vi "Button and Switch CCS.vi"() -> ()   [LabVIEW 2020]
uses:
  <vilib>/addons/control/pid/autopid.llb/PID autotuning parameters (adv).ctl
  <vilib>/addons/control/pid/pid.llb/PID Time Unit.ctl
  <vilib>/addons/control/pid/pid.llb/PID Structure.ctl
  <vilib>/addons/control/pid/pid.llb/PID Gain Unit.ctl
  <vilib>/Instr/_visa.llb/VISA Configure Serial Port (Instr).vi
  <vilib>/addons/control/pid/pid.llb/PID Structure Conversion (DBL).vi
  <vilib>/addons/control/pid/pid.llb/PID Advanced (DBL).vi
  <vilib>/addons/control/pid/NI_PID_autopid.lvlib
  <vilib>/ptbypt/NI_PtbyPt.lvlib
  <vilib>/addons/control/pid/NI_PID_pid.lvlib
panel:
  out "Image Out 2":T1(plugin-control) caption="Image Out"
  out "D":bool
  out "N":bool=TRUE
  out "R":bool
  out "P":bool
  out "PWM Previous":dbl
  in  "auto? ACC":bool
  out "Limit Setpoint":u64
  out "Limit Active":bool
  in  "Limit -":bool
  in  "Limit +":bool
  in  "Limit Speed":bool
  in  "gamma":dbl format="%.2f"
  in  "alpha":dbl=0.2 format="%.2f"
  in  "proportional unit":T2 items=["Gain (K)", "Band (PB)"]
  in  "PID structure":T3 items=["Academic (Standard)", "Parallel", "Series"]
  in  "derivative unit":T4=1 items=["min", "s"]
  in  "integral unit":T4=1 items=["min", "s"]
  in  "derivative":dbl
  in  "integral":dbl
  in  "proportional":dbl=10.0
  in  "linearity":dbl=0.9 format="%.2f"
  in  "beta":dbl=0.7 format="%.2f"
  in  "reinitialize? (F) 2":bool
  out "Speed Setpoint (km/h)":dbl
  out "Target Distance (m)":dbl
  out "Time Level":dbl=2.1
  out "Distance (m)":i8=66
  out "Brake Light":bool
  in  "VISA resource name":refnum<visa-resource-name>="COM5"
  in  "baud rate":u32=115200
  out "RPM":i64(knob) scale=0.0..650.0
  out "VELOCITY":u64(knob) scale=0.0..200.0
  out "GAS PEDAL":u8(slide) scale=0.0..255.0
  out "BRAKE PEDAL":u8(slide) scale=0.0..255.0
  out "VELOCITY":cluster{"VELOCITY":u64, "Cruise Setpoint":u64}(graph)
  in  "autotune? (F)":bool
  in  "PID gains":T5={"proportional gain (Kc)"=0.261831, "integral time (Ti, min)"=0.013639, "derivative time (Td, min)"=0.0} {"derivative time (Td, min)" format="%#.6g"; "integral time (Ti, min)" format="%#.6g"; "proportional gain (Kc)" format="%#.6g"}
  in  "dt (s)":dbl=0.02
  in  "reinitialize? (F)":bool
  in  "autotuning parameters":T6={"technique"=0, "type of controller"=1, "control specification"=0, "amplitude"=30.0} {"amplitude" format="%.2f"; "control specification" items=["normal", "fast", "slow"]; "type of controller" items=["P", "PI", "PID"]; "technique" items=["Step Open Loop", "Step Closed Loop", "Relay", "PID Relay"]}
  out "completed?":bool
  out "tuned PID gains":T5={"proportional gain (Kc)"=0.261831, "integral time (Ti, min)"=0.013639, "derivative time (Td, min)"=0.0} {"derivative time (Td, min)" format="%#.6g"; "integral time (Ti, min)" format="%#.6g"; "proportional gain (Kc)" format="%#.6g"}
  in  "auto? Speed Control":bool
  in  "ACCEPT SPEED PID":bool
  out "MOTOR CONTROL":dbl(graph)
  in  "stop":bool
  in  "PID Mode":i64(knob)=1 scale=1.0..3.0
  in  "Cruise Enable":bool
  in  "Distance":bool
  out "Distance Level":i8=4
  out "Cruise Active":bool
  out "Cruise Setpoint":u64
  in  "Speed +":bool
  in  "Speed -":bool
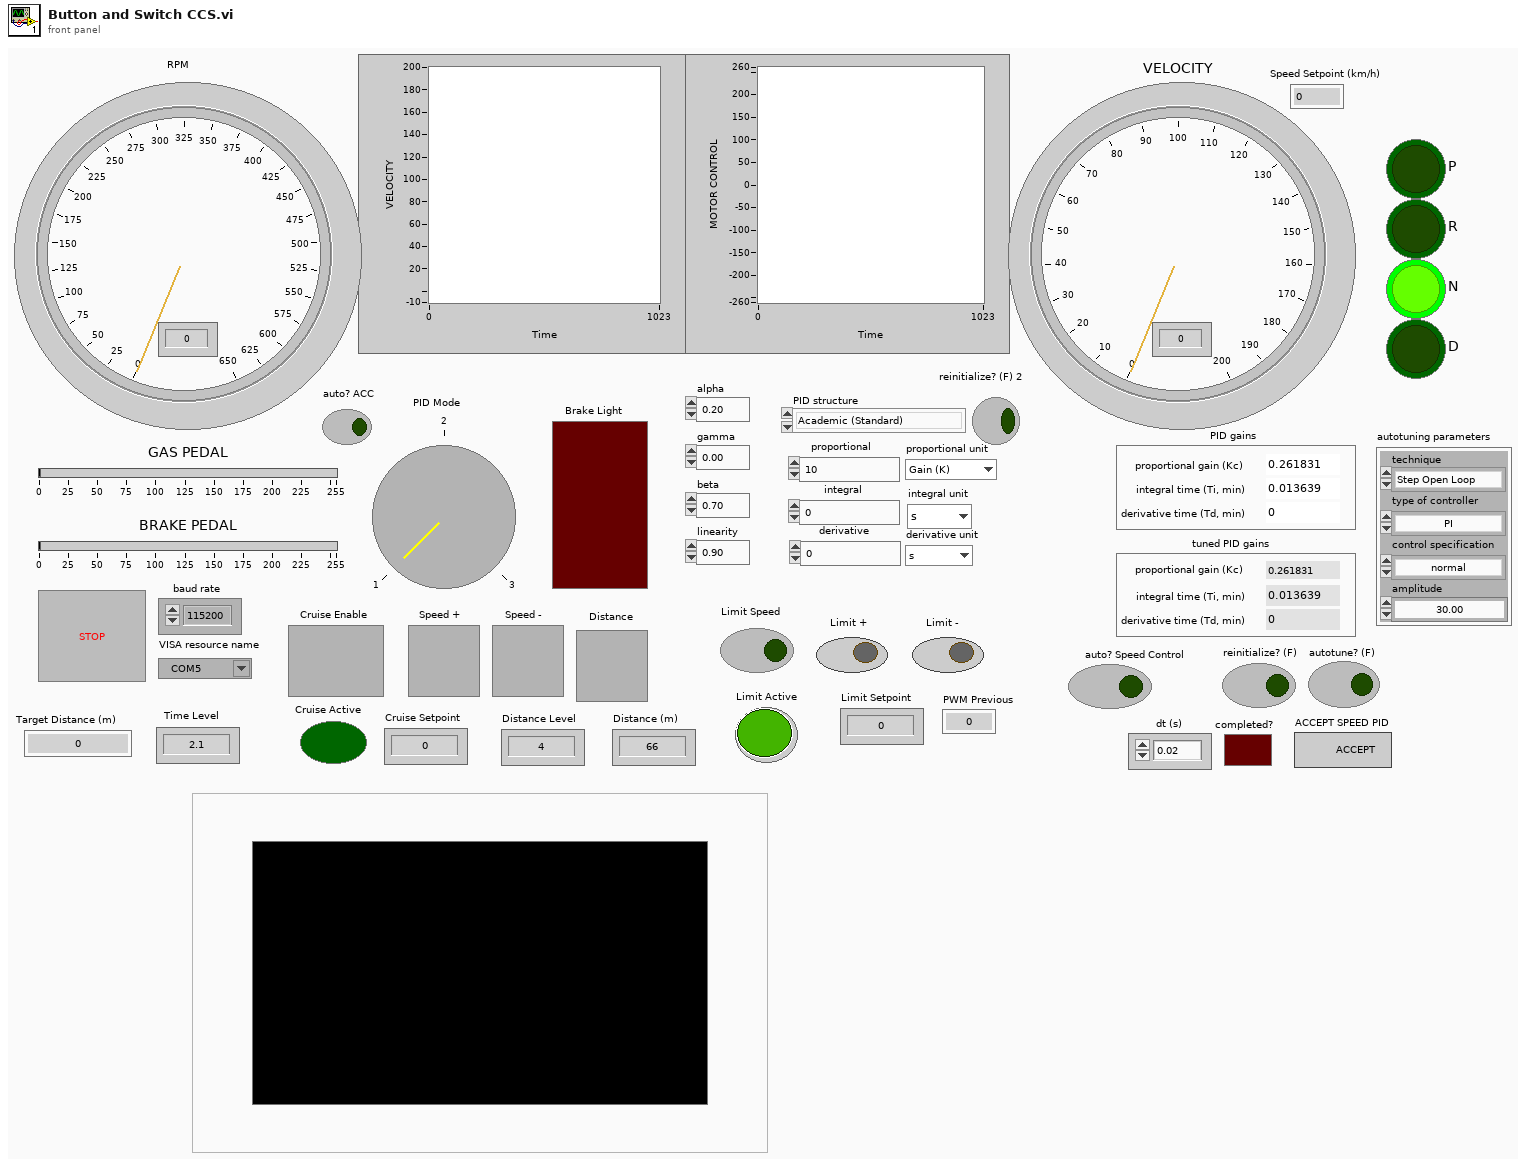
[diagram p1: front panel]
types:
  T1 = typedef "IMAQ Image.ctl" = refnum<image>
  T2 = typedef "NI_PID_pid.lvlib/PID Gain Unit.ctl" = u16
  T3 = typedef "NI_PID_pid.lvlib/PID Structure.ctl" = u16
  T4 = typedef "NI_PID_pid.lvlib/PID Time Unit.ctl" = u16
  T5 = cluster{"proportional gain (Kc)":dbl, "integral time (Ti, min)":dbl, "derivative time (Td, min)":dbl}
  T6 = typedef "NI_PID_autopid.lvlib/PID autotuning parameters (adv).ctl" = cluster{"technique":u16, "type of controller":u16, "control specification":u16, "amplitude":dbl}
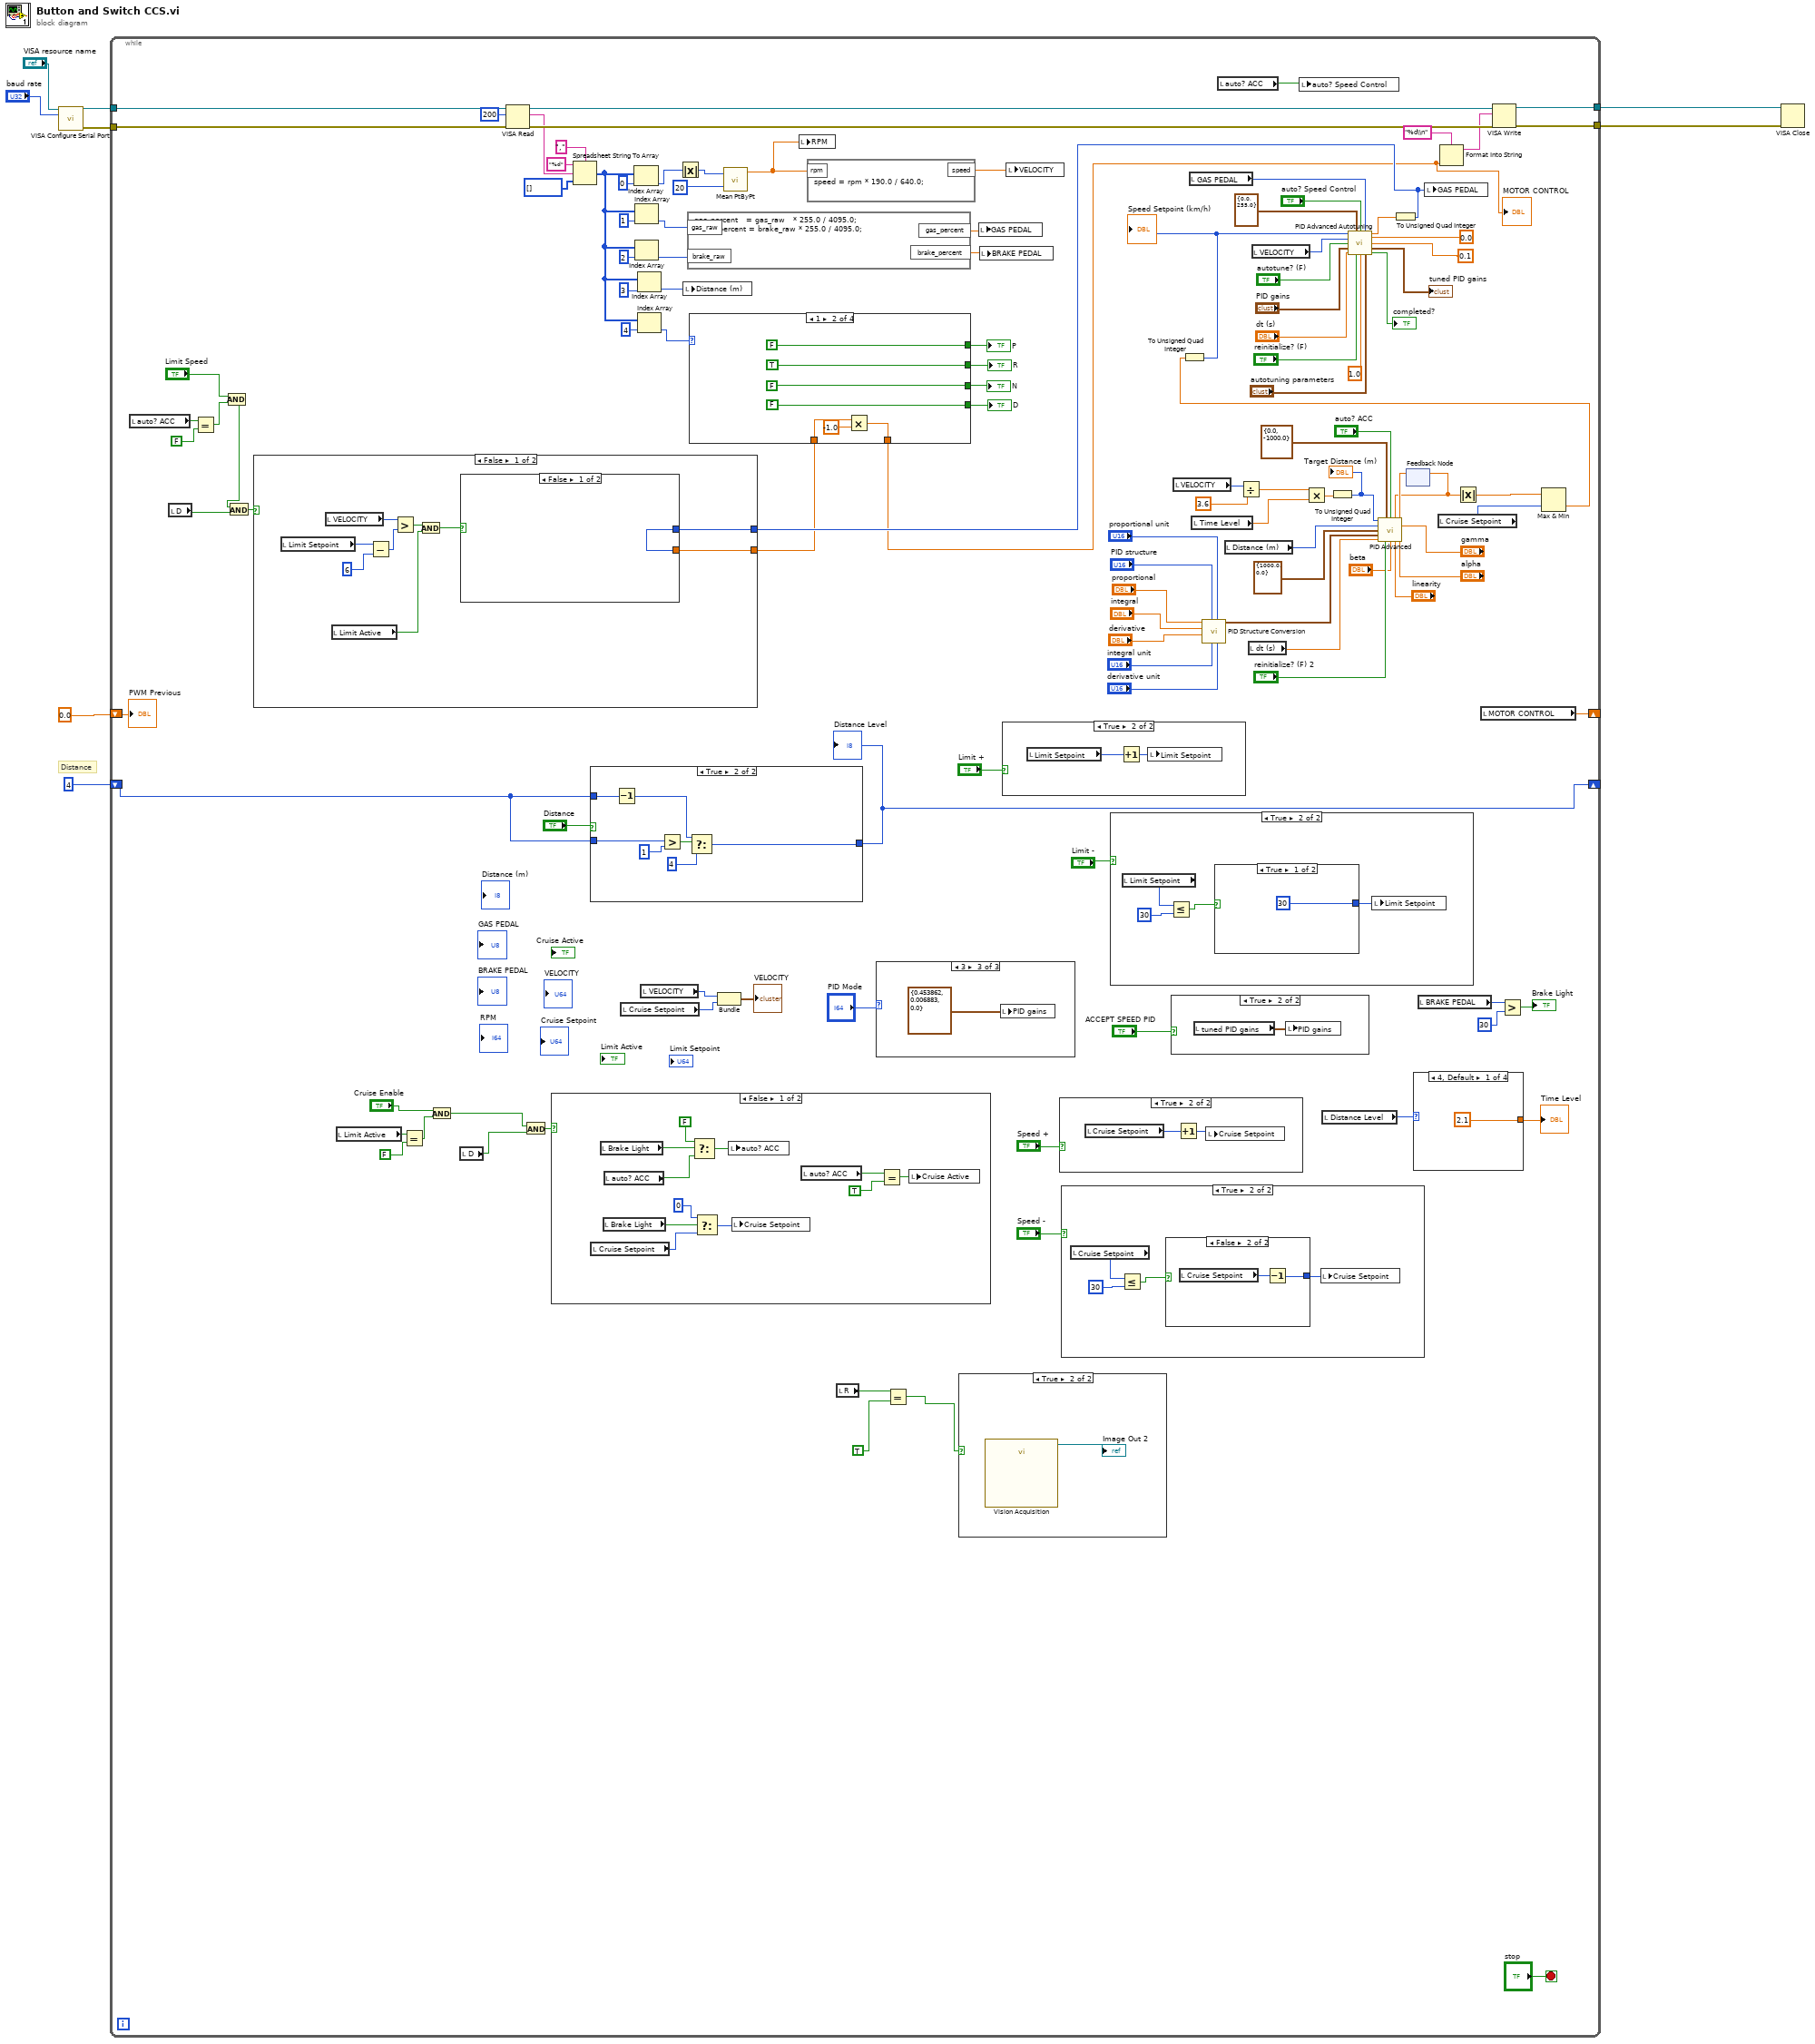
[diagram p0: block diagram]
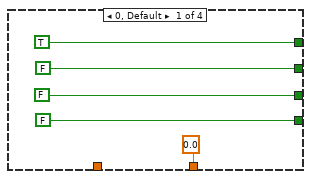
[diagram p3: hidden frame]
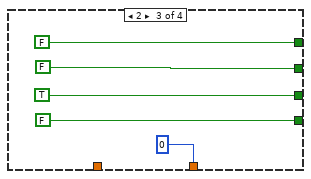
[diagram p4: hidden frame]
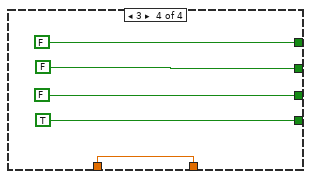
[diagram p5: hidden frame]
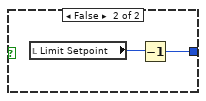
[diagram p7: hidden frame]
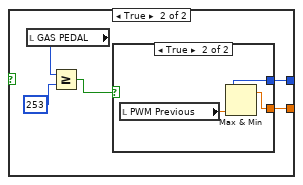
[diagram p9: hidden frame]
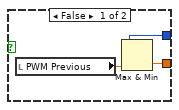
[diagram p10: hidden frame]
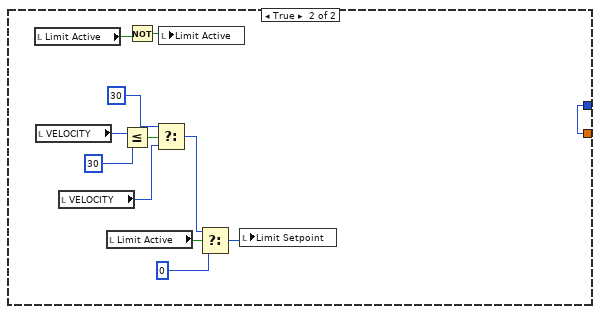
[diagram p11: hidden frame]
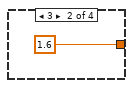
[diagram p12: hidden frame]
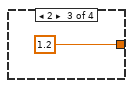
[diagram p13: hidden frame]
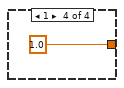
[diagram p14: hidden frame]
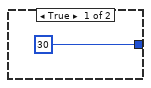
[diagram p17: hidden frame]
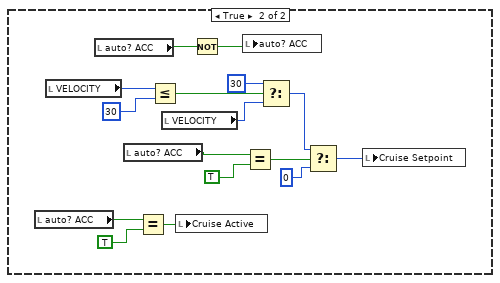
[diagram p19: hidden frame]
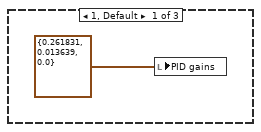
[diagram p20: hidden frame]
diagram:
  # "Distance"
  n1 = call-poly "VISA Configure Serial Port"("VISA resource name"="VISA resource name", "baud rate (9600)"="baud rate") -> ("VISA resource name out"=w7:refnum<visa-resource-name>, "error out"=w6:errorcluster)  [unwired: 12 in]
  n2 = while {
    tunnel: w7 -> [w128]
    tunnel: w6 -> [w127]
    tunnel: [w102] -> w5
    tunnel: [w103] -> w4
    shift-right: [w80] -> _
    shift-left: i64 4 ("f") -> [w81]
    shift-right: [w37] -> _
    shift-left: 0.0 ("MOTOR CONTROL") -> [w35]
    stop <- "stop" stop-if-true
    n3 = local read "auto? ACC"() -> (w41:bool)
    n4 = local read "D"() -> (w17:bool)
    n5 = Equal?(x=w41, y=FALSE) -> (x = y?=w40:bool)
    n6 = And(x="Limit Speed", y=w40) -> (x .and. y?=w18:bool)
    n7 = And(x=w18, y=w17) -> (x .and. y?=w19:bool)
    n8 = local read "Limit Active"() -> (w31:bool)
    n9 = Equal?(x=w31, y=FALSE) -> (x = y?=w32:bool)
    n10 = And(x="Cruise Enable", y=w32) -> (x .and. y?=w15:bool)
    n11 = local read "D"() -> (w14:bool)
    n12 = VISA Read(VISA resource name=w128, byte count=u32 200, error in (no error)=w127) -> (VISA resource name out=w125:refnum<visa-resource-name>, read buffer=w123:string, error out=w126:errorcluster)  [unwired: 1 out]
    n13 = And(x=w15, y=w14) -> (x .and. y?=w16:bool)
    n14 = case shown="False" w16 {
      frame False {
        n15 = local read "Cruise Setpoint"() -> (w217:u64)
        n16 = local read "Brake Light"() -> (w225:bool)
        n17 = local read "Brake Light"() -> (w218:bool)
        n18 = local read "auto? ACC"() -> (w222:bool)
        n19 = Select(t=FALSE, s=w225, f=w222) -> (s? t:f=w223:bool)
        n20 = Select(t=u64 0, s=w218, f=w217) -> (s? t:f=w215:u64)
        n21 = local write "auto? ACC"(w223) -> ()
        n22 = local write "Cruise Setpoint"(w215) -> ()
        n23 = local read "auto? ACC"() -> (w220:bool)
        n24 = Equal?(x=w220, y=TRUE) -> (x = y?=w219:bool)
        n25 = local write "Cruise Active"(w219) -> ()
      }
      frame True {
        n26 = local read "auto? ACC"() -> (w233:bool)
        n27 = local read "VELOCITY"() -> (w232:u64)
        n28 = local read "auto? ACC"() -> (w241:bool)
        n29 = local read "auto? ACC"() -> (w239:bool)
        n30 = Equal?(x=w233, y=TRUE) -> (x = y?=w226:bool)
        n31 = Less Or Equal?(x=w232, y=u64 30) -> (x <= y?=w230:bool)
        n32 = local read "VELOCITY"() -> (w229:u64)
        n33 = local write "Cruise Active"(w226) -> ()
        n34 = Not(x=w241) -> (.not. x?=w240:bool)
        n35 = local write "auto? ACC"(w240) -> ()
        n36 = Equal?(x=w239, y=TRUE) -> (x = y?=w237:bool)
        n37 = Select(t=u64 30, s=w230, f=w229) -> (s? t:f=w227:u64)
        n38 = Select(t=w227, s=w237, f=i64 0) -> (s? t:f=w236:u64)
        n39 = local write "Cruise Setpoint"(w236) -> ()
      }
    }
    n40 = Spreadsheet String To Array(delimiter (Tab)=",", format string="%d", spreadsheet string=w123, array type (2D Dbl)=i32[] []) -> (array=w26:i32[])
    n41 = case shown="True" "Distance" {
      tunnel: w81 -> [w198 w205]
      tunnel: w81 -> [_ w204]
      tunnel: [w198 w199] -> w80
      frame False {
      }
      frame True {
        n42 = Decrement(x=w205) -> (x-1=w201:i64)
        n43 = Greater?(x=w204, y=i64 1) -> (0:w202:bool)
        n44 = Select(t=w201, s=w202, f=i64 4) -> (s? t:f=w199:i64)
      }
    }
    "Distance Level" <- w80
    n45 = local read "Cruise Setpoint"() -> (w85:u64)
    n46 = Index Array(array=w26, index=0) -> (element=w96:i32)
    n47 = Index Array(array=w26, index=1) -> (element=w99:i32)
    n48 = Index Array(array=w26, index=2) -> (element=w98:i32)
    n49 = Index Array(array=w26, index=3) -> (element=w75:i32)
    n50 = Index Array(array=w26, index=4) -> (element=w24:i32)
    n51 = local read "VELOCITY"() -> (w91:u64)
    n52 = Absolute Value(x=w96) -> (abs(x)=w95:i32)
    n53 = local write "Distance (m)"(w75) -> ()
    n54 = formula code="gas_percent   = gas_raw   * 255.0 / 4095.0;\nbrake_percent = brake_raw * 255.0 / 4095.0;"("gas_raw"=w99, "brake_raw"=w98) -> ("gas_percent"=w34:dbl, "brake_percent"=w97:dbl)
    n55 = Bundle("VELOCITY"=w91, "Cruise Setpoint"=w85) -> (→"VELOCITY":cluster{"VELOCITY":u64, "Cruise Setpoint":u64})  [unwired: 1 in]
    n56 = call <vilib>:"Mean PtByPt.vi"("x"=w95, "sample length"=20) -> ("mean"=w100:dbl)  [unwired: 2 in, 1 out]
    n57 = local write "RPM"(w100) -> ()
    n58 = formula code="speed = rpm * 190.0 / 640.0;"("rpm"=w100) -> ("speed"=w101:dbl)
    n59 = local read "R"() -> (w11:bool)
    n60 = case shown="3" "PID Mode" {
      frame 1, Default {
        n61 = local write "PID gains"(T5 {"proportional gain (Kc)"=0.261831, "integral time (Ti, min)"=0.013639, "derivative time (Td, min)"=0.0} ("PID gains")) -> ()
      }
      frame 2 {
        n62 = local write "PID gains"(T5 {"proportional gain (Kc)"=0.638776, "integral time (Ti, min)"=0.011721, "derivative time (Td, min)"=0.0} ("PID gains")) -> ()
      }
      frame 3 {
        n63 = local write "PID gains"(T5 {"proportional gain (Kc)"=0.453862, "integral time (Ti, min)"=0.006883, "derivative time (Td, min)"=0.0} ("PID gains")) -> ()
      }
    }
    n64 = Equal?(x=w11, y=TRUE) -> (x = y?=w9:bool)
    n65 = case shown="True" w9 {
      frame False {
      }
      frame True {
        n66 = call "Vision Acquisition"() -> ("Image Out"=→"Image Out 2":T1)  [unwired: 23 in, 4 out]
      }
    }
    n67 = local write "GAS PEDAL"(w34) -> ()
    n68 = local write "BRAKE PEDAL"(w97) -> ()
    n69 = case shown="True" "Limit +" {
      frame False {
      }
      frame True {
        n70 = local read "Limit Setpoint"() -> (w160:u64)
        n71 = Increment(x=w160) -> (x+1=w159:u64)
        n72 = local write "Limit Setpoint"(w159) -> ()
      }
    }
    n73 = local write "VELOCITY"(w101) -> ()
    n74 = case shown="True" "Speed +" {
      frame False {
      }
      frame True {
        n75 = local read "Cruise Setpoint"() -> (w213:u64)
        n76 = Increment(x=w213) -> (x+1=w214:u64)
        n77 = local write "Cruise Setpoint"(w214) -> ()
      }
    }
    n78 = case shown="True" "Speed -" {
      frame False {
      }
      frame True {
        n79 = local read "Cruise Setpoint"() -> (w208:u64)
        n80 = Less Or Equal?(x=w208, y=u64 30) -> (x <= y?=w206:bool)
        n81 = case shown="False" w206 {
          tunnel: [u64 30 ("y") w211] -> w209
          frame True {
          }
          frame False {
            n82 = local read "Cruise Setpoint"() -> (w212:u64)
            n83 = Decrement(x=w212) -> (x-1=w211:u64)
          }
        }
        n84 = local write "Cruise Setpoint"(w209) -> ()
      }
    }
    n85 = case shown="True" "Limit -" {
      frame False {
      }
      frame True {
        n86 = local read "Limit Setpoint"() -> (w154:u64)
        n87 = Less Or Equal?(x=w154, y=u64 30) -> (x <= y?=w152:bool)
        n88 = case shown="True" w152 {
          tunnel: [u64 30 ("y") w157] -> w155
          frame True {
          }
          frame False {
            n89 = local read "Limit Setpoint"() -> (w158:u64)
            n90 = Decrement(x=w158) -> (x-1=w157:u64)
          }
        }
        n91 = local write "Limit Setpoint"(w155) -> ()
      }
    }
    n92 = case shown="True" "ACCEPT SPEED PID" {
      frame False {
      }
      frame True {
        n93 = local read "tuned PID gains"() -> (w245:T5)
        n94 = local write "PID gains"(w245) -> ()
      }
    }
    n95 = local read "VELOCITY"() -> (w69:u64)
    n96 = local read "GAS PEDAL"() -> (w86:u8)
    n97 = local read "Time Level"() -> (w70:dbl)
    n98 = call-poly <vilib>:"PID Structure Conversion.vi"("derivative unit"="derivative unit", "proportional unit"="proportional unit", "integral unit"="integral unit", "PID structure"="PID structure", "derivative"="derivative", "integral"="integral", "proportional"="proportional") -> ("PID gains"=w46:T5)  [unwired: 4 in]
    n99 = local read "auto? ACC"() -> (w42:bool)
    n100 = local read "Distance (m)"() -> (w68:i8)
    n101 = Divide(x=w69, y=3.6) -> (x/y=w71:dbl)
    n102 = local read "dt (s)"() -> (w62:dbl)
    n103 = local read "VELOCITY"() -> (w114:u64)
    n104 = local write "auto? Speed Control"(w42) -> ()
    n105 = Multiply(x=w71, y=w70) -> (x*y=w57:dbl)
    n106 = local read "Distance Level"() -> (w74:i8)
    n107 = To Unsigned Quad Integer(1:w57) -> (0:w56:u64)
    "Target Distance (m)" <- w56
    n108 = feedback #1() -> (w61:dbl)  [unwired: 1 in]
    n109 = call-poly <vilib>:"PID Advanced.vi"("setpoint"=w56, "output range"=cluster{"output high":dbl, "output low":dbl} {"output high"=0.0, "output low"=-1000.0}, "auto? (T)"="auto? ACC", "manual control"=w61, "process variable"=w68, "gamma"="gamma", "setpoint range"=cluster{"setpoint high":dbl, "setpoint low":dbl} {"setpoint high"=1000.0, "setpoint low"=0.0}, "alpha"="alpha", "PID gains"=w46, "dt (s)"=w62, "reinitialize? (F)"="reinitialize? (F) 2", "beta"="beta", "linearity"="linearity") -> ("output"=w63:dbl)  [unwired: 1 in, 1 out]
    n110 = feedback-in #1(w63) -> ()
    n111 = case shown="4, Default" w74 {
      tunnel: [2.1 ("Time Level") 1.6 ("Time Level") 1.2 ("Time Level") 1.0 ("Time Level")] -> w73
      frame 4, Default {
      }
      frame 3 {
      }
      frame 2 {
      }
      frame 1 {
      }
    }
    "Time Level" <- w73
    n112 = local read "BRAKE PEDAL"() -> (w79:u8)
    n113 = local read "Cruise Setpoint"() -> (w65:u64)
    n114 = Absolute Value(x=w61) -> (abs(x)=w60:dbl)
    n115 = local read "MOTOR CONTROL"() -> (w37:dbl)
    n116 = Greater?(x=w79, y=u8 30) -> (0:→"Brake Light":bool)
    n117 = Max & Min(x=w60, y=w65) -> (min(x,y)=w54:dbl)  [unwired: 1 out]
    n118 = To Unsigned Quad Integer(1:w54) -> (0:w55:u64)
    "Speed Setpoint (km/h)" <- w55
    n119 = call <vilib>:"PID Advanced Autotuning.vi"("setpoint"=w55, "output range"=cluster{"output high":dbl, "output low":dbl} {"output high"=0.0, "output low"=255.0}, "auto? (F)"="auto? Speed Control", "manual control"=w86, "process variable"=w114, "gamma"=0.0, "autotune? (F)"="autotune? (F)", "alpha"=0.1, "PID gains"="PID gains", "dt (s)"="dt (s)", "reinitialize? (F)"="reinitialize? (F)", "beta"=1.0, "autotuning parameters"="autotuning parameters") -> ("output"=w28:dbl, "tuned PID gains"=→"tuned PID gains":T5, "tuning completed?"=→"completed?":bool)
    n120 = To Unsigned Quad Integer(1:w28) -> (0:w27:u64)
    n121 = case shown="False" w19 {
      tunnel: w27 -> [w168 w182]
      tunnel: [w167 w182] -> w13
      frame False {
        n122 = local read "Limit Setpoint"() -> (w162:u64)
        n123 = local read "VELOCITY"() -> (w169:u64)
        n124 = local read "Limit Active"() -> (w165:bool)
        n125 = Subtract(x=w162, y=u64 6) -> (x-y=w163:u64)
        n126 = Greater?(x=w169, y=w163) -> (0:w166:bool)
        n127 = And(x=w166, y=w165) -> (x .and. y?=w164:bool)
        n128 = case shown="False" w164 {
          tunnel: w168 -> [w170 w175]
          tunnel: [w170 w174] -> w167
          frame False {
          }
          frame True {
            n129 = local read "GAS PEDAL"() -> (w173:u8)
            n130 = Greater Or Equal?(x=w173, y=u8 253) -> (x >= y?=w171:bool)
            n131 = case shown="True" w171 {
              tunnel: w175 -> [w177 w180]
              tunnel: [w176 w179] -> w174
              frame False {
                n132 = local read "PWM Previous"() -> (w178:dbl)
                n133 = Max & Min(x=w177, y=w178) -> (min(x,y)=w176:dbl)  [unwired: 1 out]
              }
              frame True {
                n134 = local read "PWM Previous"() -> (w181:dbl)
                n135 = Max & Min(x=w180, y=w181) -> (max(x,y)=w179:dbl)  [unwired: 1 out]
              }
            }
          }
        }
      }
      frame True {
        n136 = local read "Limit Active"() -> (w187:bool)
        n137 = local read "VELOCITY"() -> (w193:u64)
        n138 = local read "VELOCITY"() -> (w190:u64)
        n139 = local read "Limit Active"() -> (w186:bool)
        n140 = Less Or Equal?(x=w193, y=u64 30) -> (x <= y?=w191:bool)
        n141 = Not(x=w187) -> (.not. x?=w188:bool)
        n142 = Select(t=u64 30, s=w191, f=w190) -> (s? t:f=w185:u64)
        n143 = local write "Limit Active"(w188) -> ()
        n144 = Select(t=w185, s=w186, f=u64 0) -> (s? t:f=w183:u64)
        n145 = local write "Limit Setpoint"(w183) -> ()
      }
    }
    n146 = case shown="1" w24 {
      tunnel: [FALSE ("D") FALSE ("D") FALSE ("D") TRUE ("D")] -> w23
      tunnel: [FALSE ("N") FALSE ("N") TRUE ("N") FALSE ("N")] -> w22
      tunnel: [FALSE ("R") TRUE ("R") FALSE ("R") FALSE ("R")] -> w21
      tunnel: [TRUE ("P") FALSE ("P") FALSE ("P") FALSE ("P")] -> w20
      tunnel: w13 -> [_ w137 _ w147]
      tunnel: [0.0 ("index") w136 0 ("index") w147] -> w12
      frame 0, Default {
      }
      frame 1 {
        n147 = Multiply(x=w137, y=-1.0) -> (x*y=w136:dbl)
      }
      frame 2 {
      }
      frame 3 {
      }
    }
    "MOTOR CONTROL" <- w12
    "P" <- w20
    "R" <- w21
    "N" <- w22
    "D" <- w23
    n148 = local write "GAS PEDAL"(w27) -> ()
    n149 = Format Into String(format string="%d\\n", w12) -> (resulting string=w115:string)  [unwired: 2 in, 1 out]
    n150 = VISA Write(VISA resource name=w125, write buffer=w115, error in (no error)=w126) -> (VISA resource name out=w103:refnum<visa-resource-name>, error out=w102:errorcluster)  [unwired: 1 out]
    "PWM Previous" <- w35
  }
  n151 = VISA Close(VISA resource name=w4, error in (no error)=w5) -> ()  [unwired: 1 out]
